vi "send&receive_TestSuite.vi"() -> ()   [LabVIEW 2018, in "LV2Julia_examples.lvlib"]
uses:
  LV2Julia_examples.lvlib
  LV2Julia_core/VIs/Server or client state.ctl
  LV2Julia_core/VIs/detailed error info.ctl
  LV2Julia_core/VIs/StackFrame.ctl
  LV2Julia_core/VIs/Numeric Types enum.ctl
  LV2Julia_core/VIs/Commands.ctl
  LV2Julia_core/VIs/commands LV2Jl.ctl
  0f3c6ff9-6efb-4048-9743-f0faf74ba571.vi
  a0325a13-fabe-4ce2-9e5f-cb47086c548e.vi
  7f01987e-74d6-4a03-8747-02f9f83a463d.vi
  79db7e0a-da4c-4117-a634-db979a193aea.vi
  99f1ef0e-755f-4741-8b5d-28859cadfccc.vi
  28f6b6a8-06e1-472c-a07e-67bcf9cc4e65.vi
  f8b325f9-9a1a-4df1-afd8-c5f3d250536f.vi
  a48dd356-bbba-47e0-9e2d-40331a29731c.vi
  80a357a5-d281-45e5-bb39-cf6b9d5a1e33.vi
  f79ed0ed-9efb-49b8-8cfa-ee86261ff89e.vi
  9cb09b36-286d-49e3-8dd2-a7b0f5b1e9d8.vi
  1a7f9d96-89a5-4905-829b-2a4edb26e723.vi
  cfafe85d-2515-4c22-937f-8121ed6e9d54.vi
  d2cb43a9-9305-42fb-ad58-bce983510195.vi
  0f3c6ff9-6efb-4048-9743-f0faf74ba571.vi/c050a881-ebb0-4e81-b48e-5d54ac6d298c.vi
  0f3c6ff9-6efb-4048-9743-f0faf74ba571.vi/f138d779-8015-4f82-8c48-da5c27a321f7.vi
  0f3c6ff9-6efb-4048-9743-f0faf74ba571.vi/6f5853da-1522-42ed-a631-8137277f6bd0.vi
  0f3c6ff9-6efb-4048-9743-f0faf74ba571.vi/334a13bf-ed79-421d-8f9d-442316ab956b.vi
  0f3c6ff9-6efb-4048-9743-f0faf74ba571.vi/8f08bb46-79c7-4cf6-8c43-e5292f35a42a.vi
  a0325a13-fabe-4ce2-9e5f-cb47086c548e.vi/0a023b70-b2b7-4b51-b4a8-1637e8f72752.vi
  a0325a13-fabe-4ce2-9e5f-cb47086c548e.vi/abfddf90-bad1-40a2-8341-74545abc888a.vi
  a0325a13-fabe-4ce2-9e5f-cb47086c548e.vi/e109d5e2-aea3-4de8-91e8-3aff7ff5e1a5.vi
  a0325a13-fabe-4ce2-9e5f-cb47086c548e.vi/2119aad2-e76b-4395-bc38-e2441a866829.vi
  a0325a13-fabe-4ce2-9e5f-cb47086c548e.vi/bbe2ee9c-aeb3-4e4f-93f8-3db8855d79ac.vi
  7f01987e-74d6-4a03-8747-02f9f83a463d.vi/bf06bc0c-d54c-4899-bc86-944563b4b303.vi
  7f01987e-74d6-4a03-8747-02f9f83a463d.vi/d4eb1beb-9046-40bb-82cb-9c8078805344.vi
  7f01987e-74d6-4a03-8747-02f9f83a463d.vi/5686e550-6946-4fb3-9876-dc3418ab0293.vi
  7f01987e-74d6-4a03-8747-02f9f83a463d.vi/ffdc1569-392d-4031-a554-eaded28feac0.vi
  7f01987e-74d6-4a03-8747-02f9f83a463d.vi/e28b746a-5d22-4361-bc60-6e965f2af8e6.vi
  79db7e0a-da4c-4117-a634-db979a193aea.vi/5c498217-6613-458c-8874-fa92d6c19748.vi
  79db7e0a-da4c-4117-a634-db979a193aea.vi/90651d55-7251-4542-bf1a-96215a5cb46c.vi
  79db7e0a-da4c-4117-a634-db979a193aea.vi/4ea0e9b0-802e-4012-92bd-3a6280912451.vi
  99f1ef0e-755f-4741-8b5d-28859cadfccc.vi/ccb71516-df13-49fa-b0f6-e0b8672de1da.vi
  99f1ef0e-755f-4741-8b5d-28859cadfccc.vi/34444bcf-5933-4351-bbc5-1eae9a0680b0.vi
  99f1ef0e-755f-4741-8b5d-28859cadfccc.vi/000cc600-1167-4cf4-928d-6ab7aa667d42.vi
  99f1ef0e-755f-4741-8b5d-28859cadfccc.vi/98e98eea-062a-4f87-a790-41d557d372ce.vi
  99f1ef0e-755f-4741-8b5d-28859cadfccc.vi/eb945e44-4973-4a99-b8fc-568457e51597.vi
  28f6b6a8-06e1-472c-a07e-67bcf9cc4e65.vi/09974be2-1a4f-442e-861e-99198c07ad3e.vi
  28f6b6a8-06e1-472c-a07e-67bcf9cc4e65.vi/d0db5e8f-3a3c-4f1f-98d6-975ebc25a533.vi
  28f6b6a8-06e1-472c-a07e-67bcf9cc4e65.vi/c2a43064-5d3e-4f07-a41e-f48ba3bb7a5d.vi
  28f6b6a8-06e1-472c-a07e-67bcf9cc4e65.vi/cb57ac50-2f4d-40c6-84c3-4b337ccbba5c.vi
  28f6b6a8-06e1-472c-a07e-67bcf9cc4e65.vi/ce760082-6063-416a-be6f-af541c50d0f9.vi
  f8b325f9-9a1a-4df1-afd8-c5f3d250536f.vi/d0a21f22-daf0-459d-8dea-c9de37d976a3.vi
  f8b325f9-9a1a-4df1-afd8-c5f3d250536f.vi/3938edcc-9689-4aa2-8890-51d0be5f89a6.vi
  f8b325f9-9a1a-4df1-afd8-c5f3d250536f.vi/ea9f557a-cbf4-4eb9-9afd-8566b7af0bf0.vi
  f8b325f9-9a1a-4df1-afd8-c5f3d250536f.vi/f50092b0-9f6c-4b67-b069-c79229ff8c92.vi
  f8b325f9-9a1a-4df1-afd8-c5f3d250536f.vi/d586cd56-0096-4f37-b8fb-3a75e4053398.vi
  a48dd356-bbba-47e0-9e2d-40331a29731c.vi/60485b63-9fa3-41d8-b025-f222c2d1e954.vi
  a48dd356-bbba-47e0-9e2d-40331a29731c.vi/0163ca4a-c9bf-4356-9374-5b2f1cd8c8a4.vi
  a48dd356-bbba-47e0-9e2d-40331a29731c.vi/cdf03f06-3cc5-4344-93be-09e3c2b5fad7.vi
  a48dd356-bbba-47e0-9e2d-40331a29731c.vi/9e91637f-31fa-49b3-9c25-505779283418.vi
  a48dd356-bbba-47e0-9e2d-40331a29731c.vi/a6edc50e-f715-450b-aaf1-fcba25539407.vi
  80a357a5-d281-45e5-bb39-cf6b9d5a1e33.vi/4a5881ab-1715-4bbe-9af8-2363ce582ba4.vi
  80a357a5-d281-45e5-bb39-cf6b9d5a1e33.vi/b95eb402-4789-4c76-85b7-fbdb598d54ac.vi
  80a357a5-d281-45e5-bb39-cf6b9d5a1e33.vi/1290ab50-9fc8-4350-9e5d-3eaedcb8adb4.vi
  80a357a5-d281-45e5-bb39-cf6b9d5a1e33.vi/25ba802a-e149-482c-ab2a-a4ec831a7ccd.vi
  80a357a5-d281-45e5-bb39-cf6b9d5a1e33.vi/46001291-25fa-4f3c-9091-6cb6f22db868.vi
  f79ed0ed-9efb-49b8-8cfa-ee86261ff89e.vi/3667ecba-1e4f-48f0-93f6-750241537af3.vi
  f79ed0ed-9efb-49b8-8cfa-ee86261ff89e.vi/099a3fa0-6d4e-42af-8655-f73d0e4a363a.vi
  f79ed0ed-9efb-49b8-8cfa-ee86261ff89e.vi/1be80b05-b2d8-4daf-8502-32be035b1a56.vi
  f79ed0ed-9efb-49b8-8cfa-ee86261ff89e.vi/01dbd68c-7ff6-4de3-9551-88d27b9349fc.vi
  f79ed0ed-9efb-49b8-8cfa-ee86261ff89e.vi/d0bca59b-d26b-4ea8-bc33-01712e7e045f.vi
  9cb09b36-286d-49e3-8dd2-a7b0f5b1e9d8.vi/cfaefed5-3f29-4c43-88dd-88c8fc82987c.vi
  9cb09b36-286d-49e3-8dd2-a7b0f5b1e9d8.vi/62ff6e0a-46cc-460d-9e84-467dd4467122.vi
  9cb09b36-286d-49e3-8dd2-a7b0f5b1e9d8.vi/bc301213-06cb-494c-a645-9c5eb5ccddf2.vi
  9cb09b36-286d-49e3-8dd2-a7b0f5b1e9d8.vi/e85f0252-b661-475b-8e20-7d78206805a9.vi
  9cb09b36-286d-49e3-8dd2-a7b0f5b1e9d8.vi/e3c6487d-5533-439a-972b-ff6e78f91a0f.vi
  1a7f9d96-89a5-4905-829b-2a4edb26e723.vi/057b0a30-89eb-4b99-9a94-261e0d1b69db.vi
  1a7f9d96-89a5-4905-829b-2a4edb26e723.vi/1be28d80-beb7-4371-90e4-946dee281c8c.vi
  1a7f9d96-89a5-4905-829b-2a4edb26e723.vi/3a062081-cf3a-4e63-a10a-adcd83a17c12.vi
  1a7f9d96-89a5-4905-829b-2a4edb26e723.vi/70040952-3ae0-468b-bc38-5f997367fd6f.vi
  1a7f9d96-89a5-4905-829b-2a4edb26e723.vi/69db4b1a-60c2-40fd-b347-670db0906532.vi
  cfafe85d-2515-4c22-937f-8121ed6e9d54.vi/9bad1c1b-63c8-4bce-9a14-6c192ddbd00b.vi
  cfafe85d-2515-4c22-937f-8121ed6e9d54.vi/11fa2f37-74a1-4205-9996-7863193281ff.vi
  cfafe85d-2515-4c22-937f-8121ed6e9d54.vi/07d86764-f698-4878-be38-d6e095ca1645.vi
  cfafe85d-2515-4c22-937f-8121ed6e9d54.vi/c0e3ea08-1ccb-4dcb-b733-8d3fe66c5f6f.vi
  cfafe85d-2515-4c22-937f-8121ed6e9d54.vi/1336a158-84d5-45d6-a2b2-5b90658c6328.vi
  d2cb43a9-9305-42fb-ad58-bce983510195.vi/18912dc4-b1e0-4230-8a87-9373dc369598.vi
  d2cb43a9-9305-42fb-ad58-bce983510195.vi/6312c1e7-5e2e-4310-bd4a-23119c15d3f1.vi
  d2cb43a9-9305-42fb-ad58-bce983510195.vi/9cb92e57-85ab-440f-a46b-8557216ab5dd.vi
  0f3c6ff9-6efb-4048-9743-f0faf74ba571.vi/f138d779-8015-4f82-8c48-da5c27a321f7.vi/dcaca655-459b-49bd-b29b-dd229471a558.vi
  0f3c6ff9-6efb-4048-9743-f0faf74ba571.vi/6f5853da-1522-42ed-a631-8137277f6bd0.vi/6ca8c9a2-308c-4824-adeb-58a98f4b9789.vi
  0f3c6ff9-6efb-4048-9743-f0faf74ba571.vi/334a13bf-ed79-421d-8f9d-442316ab956b.vi/c3e25d4f-3d6e-45b4-ac60-a3eac4f5d4dd.vi
  a0325a13-fabe-4ce2-9e5f-cb47086c548e.vi/abfddf90-bad1-40a2-8341-74545abc888a.vi/1d4ccc36-5df4-463a-a9dd-e871d8c5e836.vi
  a0325a13-fabe-4ce2-9e5f-cb47086c548e.vi/e109d5e2-aea3-4de8-91e8-3aff7ff5e1a5.vi/72ea6f5e-8e76-457b-9f2b-3a011e948c95.vi
  a0325a13-fabe-4ce2-9e5f-cb47086c548e.vi/2119aad2-e76b-4395-bc38-e2441a866829.vi/a15880f2-4104-4f97-a4bf-5a36a63c211d.vi
  7f01987e-74d6-4a03-8747-02f9f83a463d.vi/d4eb1beb-9046-40bb-82cb-9c8078805344.vi/f0e9f2d5-ddd8-4b96-91ce-de174306b7a9.vi
  7f01987e-74d6-4a03-8747-02f9f83a463d.vi/5686e550-6946-4fb3-9876-dc3418ab0293.vi/45224409-fc74-4a19-bc5d-04c35b5f3d3a.vi
  7f01987e-74d6-4a03-8747-02f9f83a463d.vi/ffdc1569-392d-4031-a554-eaded28feac0.vi/9cbce8f5-06a0-437b-b659-713dc5751795.vi
  79db7e0a-da4c-4117-a634-db979a193aea.vi/5c498217-6613-458c-8874-fa92d6c19748.vi/0922e35c-3983-4244-89a6-de18eb35483c.vi
  79db7e0a-da4c-4117-a634-db979a193aea.vi/90651d55-7251-4542-bf1a-96215a5cb46c.vi/23ce4379-b224-4a09-8a60-6986842fc155.vi
  79db7e0a-da4c-4117-a634-db979a193aea.vi/4ea0e9b0-802e-4012-92bd-3a6280912451.vi/5cb0fd22-39b3-4679-8848-fbd0f76a760c.vi
  99f1ef0e-755f-4741-8b5d-28859cadfccc.vi/34444bcf-5933-4351-bbc5-1eae9a0680b0.vi/9b5ee3b2-61fa-464d-b808-4ed852ba9df7.vi
  99f1ef0e-755f-4741-8b5d-28859cadfccc.vi/000cc600-1167-4cf4-928d-6ab7aa667d42.vi/729371f3-82b8-4148-8e0c-782b1393dd88.vi
  99f1ef0e-755f-4741-8b5d-28859cadfccc.vi/98e98eea-062a-4f87-a790-41d557d372ce.vi/7cea73a9-e450-4982-a850-64259969e5c4.vi
  28f6b6a8-06e1-472c-a07e-67bcf9cc4e65.vi/d0db5e8f-3a3c-4f1f-98d6-975ebc25a533.vi/c32e5faa-0551-4674-b326-206195be28cb.vi
  28f6b6a8-06e1-472c-a07e-67bcf9cc4e65.vi/c2a43064-5d3e-4f07-a41e-f48ba3bb7a5d.vi/b2b31e85-ff8a-4a11-b6da-4397c20cf58c.vi
  28f6b6a8-06e1-472c-a07e-67bcf9cc4e65.vi/cb57ac50-2f4d-40c6-84c3-4b337ccbba5c.vi/00287ef4-4dad-445f-b53f-6d398869e1f1.vi
  f8b325f9-9a1a-4df1-afd8-c5f3d250536f.vi/3938edcc-9689-4aa2-8890-51d0be5f89a6.vi/9b496619-56e3-46e5-9420-f0b2b562818d.vi
  f8b325f9-9a1a-4df1-afd8-c5f3d250536f.vi/ea9f557a-cbf4-4eb9-9afd-8566b7af0bf0.vi/c59bfabf-8824-4878-9e47-809c29df3a14.vi
  f8b325f9-9a1a-4df1-afd8-c5f3d250536f.vi/f50092b0-9f6c-4b67-b069-c79229ff8c92.vi/f21eb179-c848-459d-95dc-6ea7d11ae3e0.vi
  a48dd356-bbba-47e0-9e2d-40331a29731c.vi/0163ca4a-c9bf-4356-9374-5b2f1cd8c8a4.vi/d72399aa-8d74-4fbe-b140-3f7c8dcdc190.vi
  a48dd356-bbba-47e0-9e2d-40331a29731c.vi/cdf03f06-3cc5-4344-93be-09e3c2b5fad7.vi/030a484a-d102-49b4-9b08-46c7516c605d.vi
  a48dd356-bbba-47e0-9e2d-40331a29731c.vi/9e91637f-31fa-49b3-9c25-505779283418.vi/50726ecf-c9f1-4d31-8d96-37015bd9bd52.vi
  80a357a5-d281-45e5-bb39-cf6b9d5a1e33.vi/b95eb402-4789-4c76-85b7-fbdb598d54ac.vi/a5383ccf-8e63-4c19-8ea6-c4f731bf680f.vi
  80a357a5-d281-45e5-bb39-cf6b9d5a1e33.vi/1290ab50-9fc8-4350-9e5d-3eaedcb8adb4.vi/8e8fe23a-c37e-4fb9-bc35-54979b00683a.vi
  80a357a5-d281-45e5-bb39-cf6b9d5a1e33.vi/25ba802a-e149-482c-ab2a-a4ec831a7ccd.vi/f1769c1e-122f-4ecb-91b4-8a90a66d4ed8.vi
  f79ed0ed-9efb-49b8-8cfa-ee86261ff89e.vi/099a3fa0-6d4e-42af-8655-f73d0e4a363a.vi/8ccb3943-b745-4649-895e-cc58cd628f04.vi
  f79ed0ed-9efb-49b8-8cfa-ee86261ff89e.vi/1be80b05-b2d8-4daf-8502-32be035b1a56.vi/9ebaa59b-334c-4cc3-a2e7-5942a76866e6.vi
  f79ed0ed-9efb-49b8-8cfa-ee86261ff89e.vi/01dbd68c-7ff6-4de3-9551-88d27b9349fc.vi/70455b90-e97b-459b-985c-d87a1c5f8d27.vi
  9cb09b36-286d-49e3-8dd2-a7b0f5b1e9d8.vi/62ff6e0a-46cc-460d-9e84-467dd4467122.vi/df185cf5-c5c8-4528-bf4e-04034ca71658.vi
  9cb09b36-286d-49e3-8dd2-a7b0f5b1e9d8.vi/bc301213-06cb-494c-a645-9c5eb5ccddf2.vi/68ecb473-ff7a-4f33-a7f5-8ddef986aaf0.vi
  9cb09b36-286d-49e3-8dd2-a7b0f5b1e9d8.vi/e85f0252-b661-475b-8e20-7d78206805a9.vi/805f8906-2ac2-4943-bcc2-ce7ee6626e70.vi
  1a7f9d96-89a5-4905-829b-2a4edb26e723.vi/1be28d80-beb7-4371-90e4-946dee281c8c.vi/29c07661-3584-43cb-8413-0ad855bf1dd6.vi
  1a7f9d96-89a5-4905-829b-2a4edb26e723.vi/3a062081-cf3a-4e63-a10a-adcd83a17c12.vi/92de0394-8b0e-41a9-bbdb-0ba419639912.vi
  1a7f9d96-89a5-4905-829b-2a4edb26e723.vi/70040952-3ae0-468b-bc38-5f997367fd6f.vi/85e2adf1-435c-4f2b-9704-a4fe5359d41d.vi
  cfafe85d-2515-4c22-937f-8121ed6e9d54.vi/11fa2f37-74a1-4205-9996-7863193281ff.vi/e77d8312-4832-4633-a75f-e330979cf09b.vi
  cfafe85d-2515-4c22-937f-8121ed6e9d54.vi/07d86764-f698-4878-be38-d6e095ca1645.vi/c76a7bcb-882a-45a4-b89f-2597d2f33847.vi
  cfafe85d-2515-4c22-937f-8121ed6e9d54.vi/c0e3ea08-1ccb-4dcb-b733-8d3fe66c5f6f.vi/c3839c05-a494-4270-b8a7-0c53a6508c74.vi
  0f3c6ff9-6efb-4048-9743-f0faf74ba571.vi/f138d779-8015-4f82-8c48-da5c27a321f7.vi/dcaca655-459b-49bd-b29b-dd229471a558.vi/2309c166-be4b-4e1e-8eb3-967cc5e528c7.vi
  0f3c6ff9-6efb-4048-9743-f0faf74ba571.vi/6f5853da-1522-42ed-a631-8137277f6bd0.vi/6ca8c9a2-308c-4824-adeb-58a98f4b9789.vi/cc0f1ca1-4239-4878-a66c-6570c0dfb283.vi
  0f3c6ff9-6efb-4048-9743-f0faf74ba571.vi/334a13bf-ed79-421d-8f9d-442316ab956b.vi/c3e25d4f-3d6e-45b4-ac60-a3eac4f5d4dd.vi/ab71de19-15ae-471d-8a17-25537f6b9f7d.vi
  a0325a13-fabe-4ce2-9e5f-cb47086c548e.vi/abfddf90-bad1-40a2-8341-74545abc888a.vi/1d4ccc36-5df4-463a-a9dd-e871d8c5e836.vi/621a2642-8e80-4bc6-8a7b-f91475f6563b.vi
  a0325a13-fabe-4ce2-9e5f-cb47086c548e.vi/e109d5e2-aea3-4de8-91e8-3aff7ff5e1a5.vi/72ea6f5e-8e76-457b-9f2b-3a011e948c95.vi/d84d9467-773a-4f51-b374-34f3b45e96f8.vi
  a0325a13-fabe-4ce2-9e5f-cb47086c548e.vi/2119aad2-e76b-4395-bc38-e2441a866829.vi/a15880f2-4104-4f97-a4bf-5a36a63c211d.vi/9e7459c3-f81a-4fcd-bf47-d21a6f8ffe87.vi
  7f01987e-74d6-4a03-8747-02f9f83a463d.vi/d4eb1beb-9046-40bb-82cb-9c8078805344.vi/f0e9f2d5-ddd8-4b96-91ce-de174306b7a9.vi/6f36de78-967c-4933-b5dd-0e598d4ad331.vi
  7f01987e-74d6-4a03-8747-02f9f83a463d.vi/5686e550-6946-4fb3-9876-dc3418ab0293.vi/45224409-fc74-4a19-bc5d-04c35b5f3d3a.vi/c4da7d02-ca8d-4870-8b8b-0b3c510ded96.vi
  7f01987e-74d6-4a03-8747-02f9f83a463d.vi/ffdc1569-392d-4031-a554-eaded28feac0.vi/9cbce8f5-06a0-437b-b659-713dc5751795.vi/16954a76-b9b0-4a64-9d17-38344290d572.vi
  79db7e0a-da4c-4117-a634-db979a193aea.vi/5c498217-6613-458c-8874-fa92d6c19748.vi/0922e35c-3983-4244-89a6-de18eb35483c.vi/42b4f21c-8679-4e81-9200-b8334ca139f1.vi
  79db7e0a-da4c-4117-a634-db979a193aea.vi/90651d55-7251-4542-bf1a-96215a5cb46c.vi/23ce4379-b224-4a09-8a60-6986842fc155.vi/1d0a4c10-6ff0-4457-9a73-6ff640e2168e.vi
  79db7e0a-da4c-4117-a634-db979a193aea.vi/4ea0e9b0-802e-4012-92bd-3a6280912451.vi/5cb0fd22-39b3-4679-8848-fbd0f76a760c.vi/38b5f270-5c40-4c58-9d4f-444c3803379d.vi
  99f1ef0e-755f-4741-8b5d-28859cadfccc.vi/34444bcf-5933-4351-bbc5-1eae9a0680b0.vi/9b5ee3b2-61fa-464d-b808-4ed852ba9df7.vi/79d9312b-1957-4e85-8002-522c7c56894f.vi
  99f1ef0e-755f-4741-8b5d-28859cadfccc.vi/000cc600-1167-4cf4-928d-6ab7aa667d42.vi/729371f3-82b8-4148-8e0c-782b1393dd88.vi/94117fd3-7e95-4c61-9d4c-d51d7f218b0b.vi
  99f1ef0e-755f-4741-8b5d-28859cadfccc.vi/98e98eea-062a-4f87-a790-41d557d372ce.vi/7cea73a9-e450-4982-a850-64259969e5c4.vi/fdf70d00-e57a-4a1e-bdd4-d33344dbcdc5.vi
  28f6b6a8-06e1-472c-a07e-67bcf9cc4e65.vi/d0db5e8f-3a3c-4f1f-98d6-975ebc25a533.vi/c32e5faa-0551-4674-b326-206195be28cb.vi/0d0755cb-849f-424c-b832-95ef875b3293.vi
  28f6b6a8-06e1-472c-a07e-67bcf9cc4e65.vi/c2a43064-5d3e-4f07-a41e-f48ba3bb7a5d.vi/b2b31e85-ff8a-4a11-b6da-4397c20cf58c.vi/5bc3ebd1-2eea-4fe2-bd89-161902e93dbd.vi
  28f6b6a8-06e1-472c-a07e-67bcf9cc4e65.vi/cb57ac50-2f4d-40c6-84c3-4b337ccbba5c.vi/00287ef4-4dad-445f-b53f-6d398869e1f1.vi/604b13c5-3f03-4950-a4a6-8625370b5ea2.vi
  f8b325f9-9a1a-4df1-afd8-c5f3d250536f.vi/3938edcc-9689-4aa2-8890-51d0be5f89a6.vi/9b496619-56e3-46e5-9420-f0b2b562818d.vi/5740d471-efac-432f-8db3-bced88e252bb.vi
  f8b325f9-9a1a-4df1-afd8-c5f3d250536f.vi/ea9f557a-cbf4-4eb9-9afd-8566b7af0bf0.vi/c59bfabf-8824-4878-9e47-809c29df3a14.vi/6a753862-9d09-495d-b4f7-b2d74518f4a9.vi
  f8b325f9-9a1a-4df1-afd8-c5f3d250536f.vi/f50092b0-9f6c-4b67-b069-c79229ff8c92.vi/f21eb179-c848-459d-95dc-6ea7d11ae3e0.vi/f4d8b248-fa08-4394-b4bf-415efba63cb6.vi
  a48dd356-bbba-47e0-9e2d-40331a29731c.vi/0163ca4a-c9bf-4356-9374-5b2f1cd8c8a4.vi/d72399aa-8d74-4fbe-b140-3f7c8dcdc190.vi/704d183b-2037-459a-ade8-6df426d2bfbd.vi
  a48dd356-bbba-47e0-9e2d-40331a29731c.vi/cdf03f06-3cc5-4344-93be-09e3c2b5fad7.vi/030a484a-d102-49b4-9b08-46c7516c605d.vi/6afecd3f-41c9-48e9-a420-169fc65296cf.vi
  a48dd356-bbba-47e0-9e2d-40331a29731c.vi/9e91637f-31fa-49b3-9c25-505779283418.vi/50726ecf-c9f1-4d31-8d96-37015bd9bd52.vi/84b9b7d2-2a4f-4508-b6a4-45f87f7c3a5d.vi
  80a357a5-d281-45e5-bb39-cf6b9d5a1e33.vi/b95eb402-4789-4c76-85b7-fbdb598d54ac.vi/a5383ccf-8e63-4c19-8ea6-c4f731bf680f.vi/7a3d23f4-78d6-428f-aabb-d22b9a7765ad.vi
  80a357a5-d281-45e5-bb39-cf6b9d5a1e33.vi/1290ab50-9fc8-4350-9e5d-3eaedcb8adb4.vi/8e8fe23a-c37e-4fb9-bc35-54979b00683a.vi/8fc8ec74-8d15-4e22-bb13-3bab23306641.vi
  80a357a5-d281-45e5-bb39-cf6b9d5a1e33.vi/25ba802a-e149-482c-ab2a-a4ec831a7ccd.vi/f1769c1e-122f-4ecb-91b4-8a90a66d4ed8.vi/a6480028-143d-449f-a90d-1715e38a0322.vi
  f79ed0ed-9efb-49b8-8cfa-ee86261ff89e.vi/099a3fa0-6d4e-42af-8655-f73d0e4a363a.vi/8ccb3943-b745-4649-895e-cc58cd628f04.vi/91ad8c32-2595-463f-a00d-19f1a31a0ab9.vi
  f79ed0ed-9efb-49b8-8cfa-ee86261ff89e.vi/1be80b05-b2d8-4daf-8502-32be035b1a56.vi/9ebaa59b-334c-4cc3-a2e7-5942a76866e6.vi/d7ca76aa-8f91-40c8-a33d-e0fc436d8429.vi
  f79ed0ed-9efb-49b8-8cfa-ee86261ff89e.vi/01dbd68c-7ff6-4de3-9551-88d27b9349fc.vi/70455b90-e97b-459b-985c-d87a1c5f8d27.vi/8334b92e-6c89-421a-9a89-9393042ee175.vi
  9cb09b36-286d-49e3-8dd2-a7b0f5b1e9d8.vi/62ff6e0a-46cc-460d-9e84-467dd4467122.vi/df185cf5-c5c8-4528-bf4e-04034ca71658.vi/555e92da-38c3-4728-ae1a-7d35d47cec6d.vi
  9cb09b36-286d-49e3-8dd2-a7b0f5b1e9d8.vi/bc301213-06cb-494c-a645-9c5eb5ccddf2.vi/68ecb473-ff7a-4f33-a7f5-8ddef986aaf0.vi/2cb7f626-0a6b-40e1-a36b-1fffb410bdb6.vi
  9cb09b36-286d-49e3-8dd2-a7b0f5b1e9d8.vi/e85f0252-b661-475b-8e20-7d78206805a9.vi/805f8906-2ac2-4943-bcc2-ce7ee6626e70.vi/1a5fcff8-1e1b-4a10-8cb0-04266a3492f5.vi
  1a7f9d96-89a5-4905-829b-2a4edb26e723.vi/1be28d80-beb7-4371-90e4-946dee281c8c.vi/29c07661-3584-43cb-8413-0ad855bf1dd6.vi/274c10cc-6877-4fb6-876e-52686d1825c0.vi
  1a7f9d96-89a5-4905-829b-2a4edb26e723.vi/3a062081-cf3a-4e63-a10a-adcd83a17c12.vi/92de0394-8b0e-41a9-bbdb-0ba419639912.vi/ec3eeeb6-efa3-447e-bef4-ff225729b20e.vi
  1a7f9d96-89a5-4905-829b-2a4edb26e723.vi/70040952-3ae0-468b-bc38-5f997367fd6f.vi/85e2adf1-435c-4f2b-9704-a4fe5359d41d.vi/53a65439-65bc-4240-a9ef-cc811b2bd780.vi
  cfafe85d-2515-4c22-937f-8121ed6e9d54.vi/11fa2f37-74a1-4205-9996-7863193281ff.vi/e77d8312-4832-4633-a75f-e330979cf09b.vi/aed36081-aed2-409f-bc39-66819cd0b4c3.vi
  cfafe85d-2515-4c22-937f-8121ed6e9d54.vi/07d86764-f698-4878-be38-d6e095ca1645.vi/c76a7bcb-882a-45a4-b89f-2597d2f33847.vi/54c288f8-840e-43b8-aaff-0bb173d43f54.vi
  cfafe85d-2515-4c22-937f-8121ed6e9d54.vi/c0e3ea08-1ccb-4dcb-b733-8d3fe66c5f6f.vi/c3839c05-a494-4270-b8a7-0c53a6508c74.vi/3cadb2ed-87ca-4814-8e99-a2e720a8dfb1.vi
  0f3c6ff9-6efb-4048-9743-f0faf74ba571.vi/f138d779-8015-4f82-8c48-da5c27a321f7.vi/dcaca655-459b-49bd-b29b-dd229471a558.vi/2309c166-be4b-4e1e-8eb3-967cc5e528c7.vi/f6d3542d-cc1e-4d9d-9817-8d6bc396b8a7.vi
  0f3c6ff9-6efb-4048-9743-f0faf74ba571.vi/6f5853da-1522-42ed-a631-8137277f6bd0.vi/6ca8c9a2-308c-4824-adeb-58a98f4b9789.vi/cc0f1ca1-4239-4878-a66c-6570c0dfb283.vi/ff7285a8-522c-43fc-9d63-dac79a8fad90.vi
  0f3c6ff9-6efb-4048-9743-f0faf74ba571.vi/334a13bf-ed79-421d-8f9d-442316ab956b.vi/c3e25d4f-3d6e-45b4-ac60-a3eac4f5d4dd.vi/ab71de19-15ae-471d-8a17-25537f6b9f7d.vi/091f02b8-9279-4536-a74d-e36162d3ff9a.vi
  a0325a13-fabe-4ce2-9e5f-cb47086c548e.vi/abfddf90-bad1-40a2-8341-74545abc888a.vi/1d4ccc36-5df4-463a-a9dd-e871d8c5e836.vi/621a2642-8e80-4bc6-8a7b-f91475f6563b.vi/f9b6ac16-1dbf-42f9-a70d-5fd8ed98ba9f.vi
  a0325a13-fabe-4ce2-9e5f-cb47086c548e.vi/e109d5e2-aea3-4de8-91e8-3aff7ff5e1a5.vi/72ea6f5e-8e76-457b-9f2b-3a011e948c95.vi/d84d9467-773a-4f51-b374-34f3b45e96f8.vi/1fa9ed59-771e-41ed-bb50-82ff1c775e4b.vi
  a0325a13-fabe-4ce2-9e5f-cb47086c548e.vi/2119aad2-e76b-4395-bc38-e2441a866829.vi/a15880f2-4104-4f97-a4bf-5a36a63c211d.vi/9e7459c3-f81a-4fcd-bf47-d21a6f8ffe87.vi/04f1935c-411d-4607-b276-13542326c360.vi
  7f01987e-74d6-4a03-8747-02f9f83a463d.vi/d4eb1beb-9046-40bb-82cb-9c8078805344.vi/f0e9f2d5-ddd8-4b96-91ce-de174306b7a9.vi/6f36de78-967c-4933-b5dd-0e598d4ad331.vi/3483b618-6941-450d-853a-3dd4f80d8194.vi
  7f01987e-74d6-4a03-8747-02f9f83a463d.vi/5686e550-6946-4fb3-9876-dc3418ab0293.vi/45224409-fc74-4a19-bc5d-04c35b5f3d3a.vi/c4da7d02-ca8d-4870-8b8b-0b3c510ded96.vi/369bf8c1-16ba-47de-918f-01b187e51fbd.vi
  7f01987e-74d6-4a03-8747-02f9f83a463d.vi/ffdc1569-392d-4031-a554-eaded28feac0.vi/9cbce8f5-06a0-437b-b659-713dc5751795.vi/16954a76-b9b0-4a64-9d17-38344290d572.vi/b76e1231-7917-4139-a770-2dbef96067c6.vi
  79db7e0a-da4c-4117-a634-db979a193aea.vi/5c498217-6613-458c-8874-fa92d6c19748.vi/0922e35c-3983-4244-89a6-de18eb35483c.vi/42b4f21c-8679-4e81-9200-b8334ca139f1.vi/cdd67d70-fed5-40eb-bd55-64c7d9f8c0cd.vi
  79db7e0a-da4c-4117-a634-db979a193aea.vi/90651d55-7251-4542-bf1a-96215a5cb46c.vi/23ce4379-b224-4a09-8a60-6986842fc155.vi/1d0a4c10-6ff0-4457-9a73-6ff640e2168e.vi/b5e6a49d-e123-41cd-ae39-6a04b1010118.vi
  79db7e0a-da4c-4117-a634-db979a193aea.vi/4ea0e9b0-802e-4012-92bd-3a6280912451.vi/5cb0fd22-39b3-4679-8848-fbd0f76a760c.vi/38b5f270-5c40-4c58-9d4f-444c3803379d.vi/80dd6213-b969-49b8-828d-e6a134ffc038.vi
  99f1ef0e-755f-4741-8b5d-28859cadfccc.vi/34444bcf-5933-4351-bbc5-1eae9a0680b0.vi/9b5ee3b2-61fa-464d-b808-4ed852ba9df7.vi/79d9312b-1957-4e85-8002-522c7c56894f.vi/63dab871-5128-418b-a9d4-6181b1149ad7.vi
  99f1ef0e-755f-4741-8b5d-28859cadfccc.vi/000cc600-1167-4cf4-928d-6ab7aa667d42.vi/729371f3-82b8-4148-8e0c-782b1393dd88.vi/94117fd3-7e95-4c61-9d4c-d51d7f218b0b.vi/69c89fbf-0cd2-4258-9685-0a42dcae2355.vi
  99f1ef0e-755f-4741-8b5d-28859cadfccc.vi/98e98eea-062a-4f87-a790-41d557d372ce.vi/7cea73a9-e450-4982-a850-64259969e5c4.vi/fdf70d00-e57a-4a1e-bdd4-d33344dbcdc5.vi/a0095e46-2272-4885-97f1-c4be5742910c.vi
  28f6b6a8-06e1-472c-a07e-67bcf9cc4e65.vi/d0db5e8f-3a3c-4f1f-98d6-975ebc25a533.vi/c32e5faa-0551-4674-b326-206195be28cb.vi/0d0755cb-849f-424c-b832-95ef875b3293.vi/4bf715f5-e116-42cd-bc7a-13d076c33e15.vi
  28f6b6a8-06e1-472c-a07e-67bcf9cc4e65.vi/c2a43064-5d3e-4f07-a41e-f48ba3bb7a5d.vi/b2b31e85-ff8a-4a11-b6da-4397c20cf58c.vi/5bc3ebd1-2eea-4fe2-bd89-161902e93dbd.vi/b8763943-8b18-49e5-bcd9-5f6519a8b2c5.vi
  28f6b6a8-06e1-472c-a07e-67bcf9cc4e65.vi/cb57ac50-2f4d-40c6-84c3-4b337ccbba5c.vi/00287ef4-4dad-445f-b53f-6d398869e1f1.vi/604b13c5-3f03-4950-a4a6-8625370b5ea2.vi/1fd5b09f-ec90-4e67-91ff-e84f89ca8c25.vi
  f8b325f9-9a1a-4df1-afd8-c5f3d250536f.vi/3938edcc-9689-4aa2-8890-51d0be5f89a6.vi/9b496619-56e3-46e5-9420-f0b2b562818d.vi/5740d471-efac-432f-8db3-bced88e252bb.vi/9f0b073e-b391-4280-a90c-85d02cefbfb1.vi
  f8b325f9-9a1a-4df1-afd8-c5f3d250536f.vi/ea9f557a-cbf4-4eb9-9afd-8566b7af0bf0.vi/c59bfabf-8824-4878-9e47-809c29df3a14.vi/6a753862-9d09-495d-b4f7-b2d74518f4a9.vi/7897e5e8-eaa8-4330-bf23-fc2998fe9bb9.vi
  f8b325f9-9a1a-4df1-afd8-c5f3d250536f.vi/f50092b0-9f6c-4b67-b069-c79229ff8c92.vi/f21eb179-c848-459d-95dc-6ea7d11ae3e0.vi/f4d8b248-fa08-4394-b4bf-415efba63cb6.vi/8e058e81-a9b7-44e4-9997-a38aa5bfc02f.vi
  a48dd356-bbba-47e0-9e2d-40331a29731c.vi/0163ca4a-c9bf-4356-9374-5b2f1cd8c8a4.vi/d72399aa-8d74-4fbe-b140-3f7c8dcdc190.vi/704d183b-2037-459a-ade8-6df426d2bfbd.vi/289cce88-8c4c-435a-8e2c-a078df117b9e.vi
  a48dd356-bbba-47e0-9e2d-40331a29731c.vi/cdf03f06-3cc5-4344-93be-09e3c2b5fad7.vi/030a484a-d102-49b4-9b08-46c7516c605d.vi/6afecd3f-41c9-48e9-a420-169fc65296cf.vi/27de24e4-830a-48d0-a5fe-ff9ed3d4be87.vi
  a48dd356-bbba-47e0-9e2d-40331a29731c.vi/9e91637f-31fa-49b3-9c25-505779283418.vi/50726ecf-c9f1-4d31-8d96-37015bd9bd52.vi/84b9b7d2-2a4f-4508-b6a4-45f87f7c3a5d.vi/bc45bda0-d671-4435-853f-da6377ab6c0f.vi
  80a357a5-d281-45e5-bb39-cf6b9d5a1e33.vi/b95eb402-4789-4c76-85b7-fbdb598d54ac.vi/a5383ccf-8e63-4c19-8ea6-c4f731bf680f.vi/7a3d23f4-78d6-428f-aabb-d22b9a7765ad.vi/11c33436-193b-44c9-977d-ececd4a6ac51.vi
  80a357a5-d281-45e5-bb39-cf6b9d5a1e33.vi/1290ab50-9fc8-4350-9e5d-3eaedcb8adb4.vi/8e8fe23a-c37e-4fb9-bc35-54979b00683a.vi/8fc8ec74-8d15-4e22-bb13-3bab23306641.vi/f4fd83e8-1d8c-4823-9409-a0c4ae51a48c.vi
  80a357a5-d281-45e5-bb39-cf6b9d5a1e33.vi/25ba802a-e149-482c-ab2a-a4ec831a7ccd.vi/f1769c1e-122f-4ecb-91b4-8a90a66d4ed8.vi/a6480028-143d-449f-a90d-1715e38a0322.vi/99ca01ae-a83f-49a5-ae4a-080814a967d1.vi
  f79ed0ed-9efb-49b8-8cfa-ee86261ff89e.vi/099a3fa0-6d4e-42af-8655-f73d0e4a363a.vi/8ccb3943-b745-4649-895e-cc58cd628f04.vi/91ad8c32-2595-463f-a00d-19f1a31a0ab9.vi/0fc86a2f-760c-4000-a558-6625ae050d9c.vi
  f79ed0ed-9efb-49b8-8cfa-ee86261ff89e.vi/1be80b05-b2d8-4daf-8502-32be035b1a56.vi/9ebaa59b-334c-4cc3-a2e7-5942a76866e6.vi/d7ca76aa-8f91-40c8-a33d-e0fc436d8429.vi/a53a8712-ce2d-40f2-8719-5dedfc640ef9.vi
  f79ed0ed-9efb-49b8-8cfa-ee86261ff89e.vi/01dbd68c-7ff6-4de3-9551-88d27b9349fc.vi/70455b90-e97b-459b-985c-d87a1c5f8d27.vi/8334b92e-6c89-421a-9a89-9393042ee175.vi/474b7793-7654-4cc7-b10a-cc58eaf29e4f.vi
  9cb09b36-286d-49e3-8dd2-a7b0f5b1e9d8.vi/62ff6e0a-46cc-460d-9e84-467dd4467122.vi/df185cf5-c5c8-4528-bf4e-04034ca71658.vi/555e92da-38c3-4728-ae1a-7d35d47cec6d.vi/1ae85664-b332-44d4-867b-1d717d01f1b1.vi
  9cb09b36-286d-49e3-8dd2-a7b0f5b1e9d8.vi/bc301213-06cb-494c-a645-9c5eb5ccddf2.vi/68ecb473-ff7a-4f33-a7f5-8ddef986aaf0.vi/2cb7f626-0a6b-40e1-a36b-1fffb410bdb6.vi/525e6f11-a507-4ab5-8f44-f4f55daf67d4.vi
  9cb09b36-286d-49e3-8dd2-a7b0f5b1e9d8.vi/e85f0252-b661-475b-8e20-7d78206805a9.vi/805f8906-2ac2-4943-bcc2-ce7ee6626e70.vi/1a5fcff8-1e1b-4a10-8cb0-04266a3492f5.vi/1d7d714c-68c9-46d5-97e7-ece508b40457.vi
  1a7f9d96-89a5-4905-829b-2a4edb26e723.vi/1be28d80-beb7-4371-90e4-946dee281c8c.vi/29c07661-3584-43cb-8413-0ad855bf1dd6.vi/274c10cc-6877-4fb6-876e-52686d1825c0.vi/04a1345e-4259-4b92-a067-0273b67cbd8a.vi
  1a7f9d96-89a5-4905-829b-2a4edb26e723.vi/3a062081-cf3a-4e63-a10a-adcd83a17c12.vi/92de0394-8b0e-41a9-bbdb-0ba419639912.vi/ec3eeeb6-efa3-447e-bef4-ff225729b20e.vi/872e9e59-3680-4f22-9b9d-15434c4e78c9.vi
  1a7f9d96-89a5-4905-829b-2a4edb26e723.vi/70040952-3ae0-468b-bc38-5f997367fd6f.vi/85e2adf1-435c-4f2b-9704-a4fe5359d41d.vi/53a65439-65bc-4240-a9ef-cc811b2bd780.vi/2899dd3f-3718-40ac-92be-749708dd3abb.vi
  cfafe85d-2515-4c22-937f-8121ed6e9d54.vi/11fa2f37-74a1-4205-9996-7863193281ff.vi/e77d8312-4832-4633-a75f-e330979cf09b.vi/aed36081-aed2-409f-bc39-66819cd0b4c3.vi/3bf3b40a-782a-45e2-b8a0-653afe03bd13.vi
  cfafe85d-2515-4c22-937f-8121ed6e9d54.vi/07d86764-f698-4878-be38-d6e095ca1645.vi/c76a7bcb-882a-45a4-b89f-2597d2f33847.vi/54c288f8-840e-43b8-aaff-0bb173d43f54.vi/52b061ae-82a4-4929-86dd-60e1c67210a0.vi
  cfafe85d-2515-4c22-937f-8121ed6e9d54.vi/c0e3ea08-1ccb-4dcb-b733-8d3fe66c5f6f.vi/c3839c05-a494-4270-b8a7-0c53a6508c74.vi/3cadb2ed-87ca-4814-8e99-a2e720a8dfb1.vi/d5a0ec0b-00c1-4e11-af1d-53093ed117e4.vi
  LV2Julia_core/VIs/check ID validity.vi
  LV2Julia_core/VIs/bindata_descr to JSON.vi
  LV2Julia_core/VIs/check cluster field names.vi
  LV2Julia_core/VIs/concat JSON.vi
  LV2Julia_core/LV2Julia_core.lvlib
panel:
  out "arr dimension":i32
  out "numeric type":T1
  out "detailed error info":T2
  out "all elems OK":bool
  out "elem sent":cdb
  out "all arrays OK":bool
  in  "Stop JL-server":bool
  out "elem received":cdb
  out "numarray 3D":cdb[][][](array[numeric])
  out "numarray 2D":cdb[][](array[numeric])
  out "arrs equal":bool
  out "numarray 1D":cdb[](array[numeric]) format="%.1f"
  in  "index to return":cluster{"idx":u16[]}={"idx"=[1, 1, 1]} {"idx" min=1}
  out "Jl Server state out":T4
  out "short err code":u8
  out "final error":errorcluster
  # "add starting Jl server"
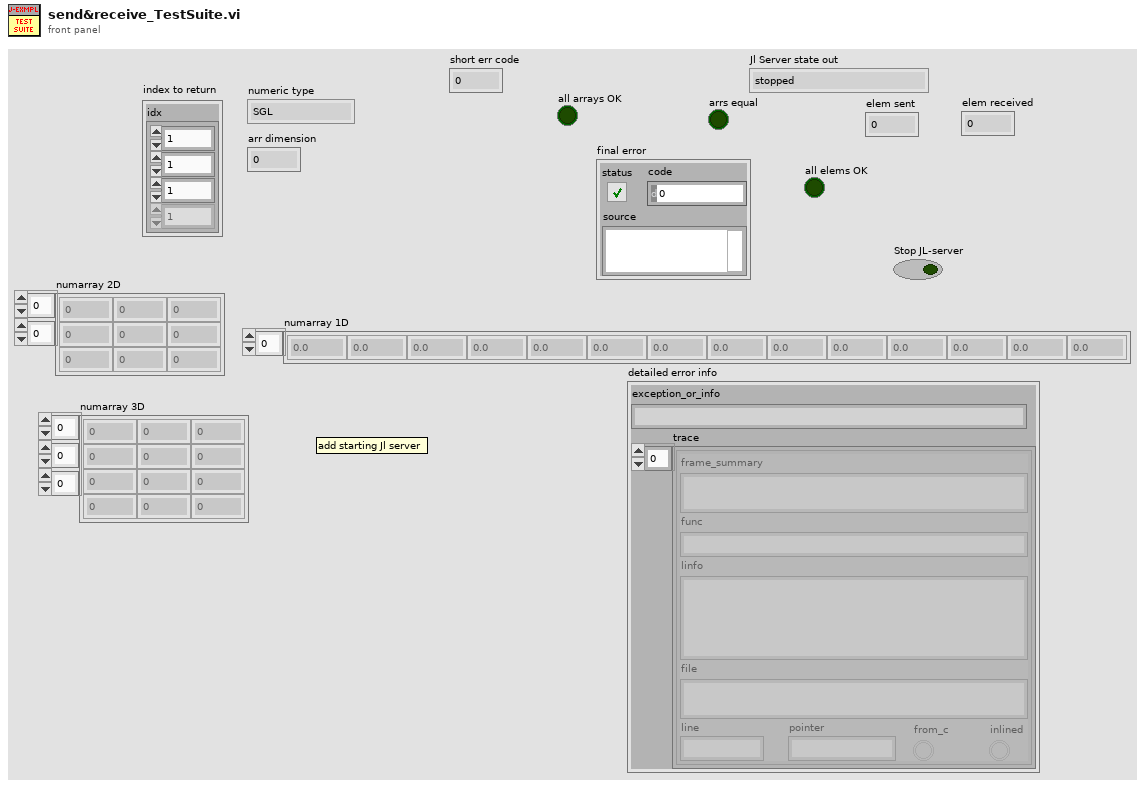
[diagram p1: front panel]
types:
  T1 = typedef "LV2Julia_core.lvlib/Numeric Types enum.ctl" = enum16{"SGL", "DBL", "I8", "I16", "I32", "I64", "U8", "U16", "U32", "U64", "CSGL", "CDBL", "boolean"}
  T2 = typedef "LV2Julia_core.lvlib/detailed error info.ctl" = cluster{"exception_or_info":string, "trace":T3[]}
  T3 = typedef "LV2Julia_core.lvlib/StackFrame.ctl" = cluster{"frame_summary":string, "func":string, "linfo":string, "file":string, "line":i32, "pointer":u64, "from_c":bool, "inlined":bool}
  T4 = typedef "LV2Julia_core.lvlib/Server or client state.ctl" = enum16{"stopped", "running", "unknown"}
  T5 = typedef "LV2Julia_core.lvlib/Commands.ctl" = enum16{"Start Jl-server & Init LV-client", "Send request & Get response ", "Stop Jl-server & Cleanup LV-client", "Cleanup LV-client", "Start Jl-server", "Stop Jl-server", "Init LV-Client", "Cleanup LV-Client", "(not allowed)", "Set LV Client state", "Set Jl Server state", "set ZMQ timeout", "read ZMQ timeout", "read-out state"}
  T6 = typedef "LV2Julia_core.lvlib/commands LV2Jl.ctl" = u8
  T7 = typedef "LV2Julia_core.lvlib/Bindata&description.ctl" = cluster{"bindata_descr":T8[], "bindata":u8[]}
  T8 = typedef "LV2Julia_core.lvlib/Bindata description.ctl" = cluster{"nofbytes":i32, "numtype":string, "start":i32, "arrdims":i32[], "kwarg_name":string, "category":string}
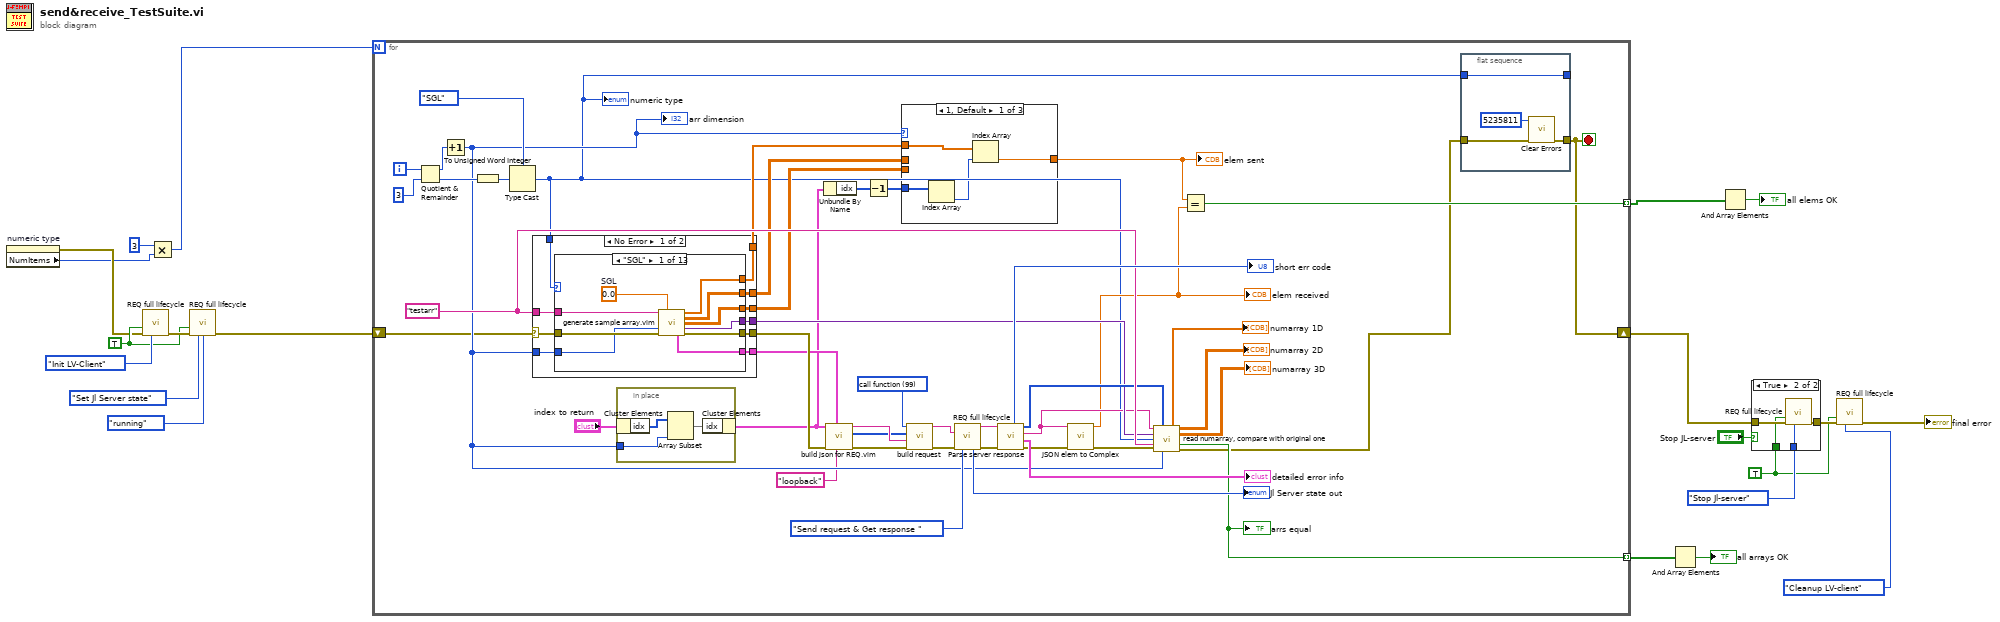
[diagram p0: block diagram]
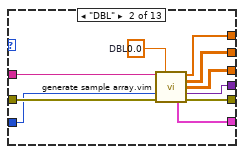
[diagram p2: hidden frame]
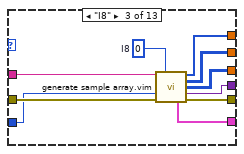
[diagram p3: hidden frame]
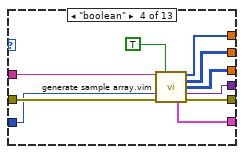
[diagram p4: hidden frame]
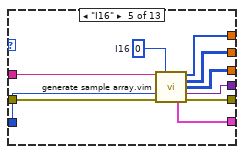
[diagram p5: hidden frame]
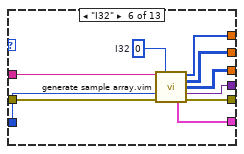
[diagram p6: hidden frame]
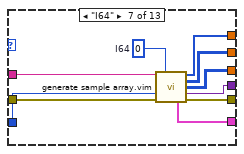
[diagram p7: hidden frame]
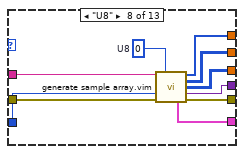
[diagram p8: hidden frame]
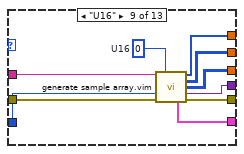
[diagram p9: hidden frame]
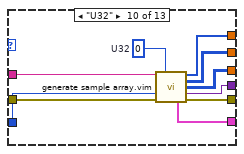
[diagram p10: hidden frame]
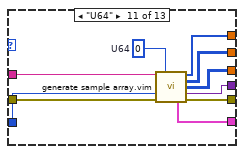
[diagram p11: hidden frame]
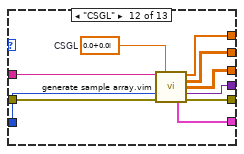
[diagram p12: hidden frame]
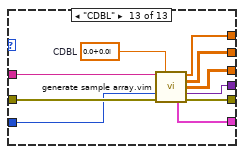
[diagram p13: hidden frame]
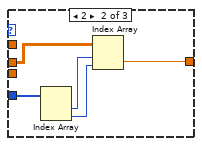
[diagram p15: hidden frame]
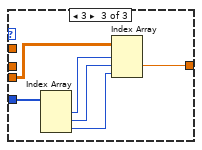
[diagram p16: hidden frame]
diagram:
  w12 = TRUE ("Force command")
  w16 = TRUE ("Force command")
  n1 = property on="numeric type" class="Enum (strict)"() -> (error out=w9:errorcluster, "NumItems"=w8:u32)  [unwired: 2 in, 1 out]
  n2 = call "REQ full lifecycle.vi"("Force command"=w12, "error in"=w9, "command"=Commands."Init LV-Client") -> ("error out"=w14:errorcluster)  [unwired: 6 in, 6 out]
  n3 = Multiply(x=u32 3, y=w8) -> (x*y=w6:u32)
  n4 = call "REQ full lifecycle.vi"("Force command"=w12, "error in"=w14, "command"=Commands."Set Jl Server state", "Jl Server state in"=Server_or_client_state."running") -> ("error out"=w3:errorcluster)  [unwired: 5 in, 6 out]
  n5 = for {
    N: w6 -> [_]
    tunnel: [w40] -> w5 mode=indexing
    shift-right: [w24] -> w21
    shift-left: w3 -> [w27]
    tunnel: [w29] -> w1 mode=indexing
    i -> [w44]
    stop <- w24 stop-if-true
    w53 = "testarr" ("Tag")
    w61 = T6 99 items=["call function"=99, "ping"=112, "stop"=115] ("Command")
    n6 = Quotient & Remainder(x=w44, y=3) -> (x-y*floor(x/y)=w36:i32, floor(x/y)=w38:i32)
    n7 = Increment(x=w36) -> (x+1=w28:i32)
    "arr dimension" <- w28
    n8 = To Unsigned Word Integer(number=w38) -> (unsigned 16bit integer=w41:u16)
    n9 = Type Cast(type=Numeric_Types_enum."SGL" ("numeric type const"), x=w41) -> (*(type *) &x=w25:T1)
    "numeric type" <- w25
    n10 = case shown="No Error" w27 {
      selector: w27 -> [w72 w212]
      tunnel: [w81 w212] -> w60
      tunnel: [w80 _] -> w59
      tunnel: w53 -> [w79 _]
      tunnel: [w78 _] -> w49
      tunnel: w25 -> [w77 _]
      tunnel: [w76 _] -> w35
      tunnel: [w75 _] -> w33
      tunnel: [w74 _] -> w32
      tunnel: w28 -> [w73 _]
      frame No Error {
        n11 = case shown="\"SGL\"" w77 {
          tunnel: [w91 w101 w111 w121 w131 w141 w151 w161 w171 w181 w191 w201 w211] -> w81
          tunnel: [w90 w100 w110 w120 w130 w140 w150 w160 w170 w180 w190 w200 w210] -> w80
          tunnel: w72 -> [w89 w99 w109 w119 w129 w139 w149 w159 w169 w179 w189 w199 w209]
          tunnel: w73 -> [w88 w98 w108 w118 w128 w138 w148 w158 w168 w178 w188 w198 w208]
          tunnel: w79 -> [w87 w97 w107 w117 w127 w137 w147 w157 w167 w177 w187 w197 w207]
          tunnel: [w85 w95 w105 w116 w125 w135 w145 w155 w165 w175 w185 w195 w205] -> w78
          tunnel: [w84 w92 w102 w113 w122 w132 w142 w152 w162 w172 w182 w192 w202] -> w74
          tunnel: [w83 w93 w103 w114 w123 w133 w143 w153 w163 w173 w183 w193 w203] -> w75
          tunnel: [w82 w94 w104 w115 w124 w134 w144 w154 w164 w174 w184 w194 w204] -> w76
          frame "SGL" {
            w86 = sgl 0.0  # SGL
            n12 = call "generate sample array.vim"("kwarg_name"=w87, "type"=w86, "dims"=w88, "error in (no error)"=w89) -> ("Array 1D"=w82:sgl[], "Array 2D"=w83:sgl[][], "Array 3D"=w84:sgl[][][], "array as variant"=w85:variant, "Bindata & descr out"=w90:T7, "error out"=w91:errorcluster)  [unwired: 5 in, 1 out]
          }
          frame "DBL" {
            w96 = 0.0  # DBL
            n13 = call "generate sample array.vim"("kwarg_name"=w97, "type"=w96, "dims"=w98, "error in (no error)"=w99) -> ("Array 1D"=w94:dbl[], "Array 2D"=w93:dbl[][], "Array 3D"=w92:dbl[][][], "array as variant"=w95:variant, "Bindata & descr out"=w100:T7, "error out"=w101:errorcluster)  [unwired: 5 in, 1 out]
          }
          frame "I8" {
            w106 = i8 0  # I8
            n14 = call "generate sample array.vim"("kwarg_name"=w107, "type"=w106, "dims"=w108, "error in (no error)"=w109) -> ("Array 1D"=w104:i8[], "Array 2D"=w103:i8[][], "Array 3D"=w102:i8[][][], "array as variant"=w105:variant, "Bindata & descr out"=w110:T7, "error out"=w111:errorcluster)  [unwired: 5 in, 1 out]
          }
          frame "boolean" {
            n15 = call "generate sample array.vim"("kwarg_name"=w117, "type"=TRUE, "dims"=w118, "error in (no error)"=w119) -> ("Array 1D"=w115:i16[], "Array 2D"=w114:i16[][], "Array 3D"=w113:i16[][][], "array as variant"=w116:variant, "Bindata & descr out"=w120:T7, "error out"=w121:errorcluster)  [unwired: 5 in, 1 out]
          }
          frame "I16" {
            w126 = i16 0  # I16
            n16 = call "generate sample array.vim"("kwarg_name"=w127, "type"=w126, "dims"=w128, "error in (no error)"=w129) -> ("Array 1D"=w124:i16[], "Array 2D"=w123:i16[][], "Array 3D"=w122:i16[][][], "array as variant"=w125:variant, "Bindata & descr out"=w130:T7, "error out"=w131:errorcluster)  [unwired: 5 in, 1 out]
          }
          frame "I32" {
            w136 = 0  # I32
            n17 = call "generate sample array.vim"("kwarg_name"=w137, "type"=w136, "dims"=w138, "error in (no error)"=w139) -> ("Array 1D"=w134:i32[], "Array 2D"=w133:i32[][], "Array 3D"=w132:i32[][][], "array as variant"=w135:variant, "Bindata & descr out"=w140:T7, "error out"=w141:errorcluster)  [unwired: 5 in, 1 out]
          }
          frame "I64" {
            w146 = i64 0  # I64
            n18 = call "generate sample array.vim"("kwarg_name"=w147, "type"=w146, "dims"=w148, "error in (no error)"=w149) -> ("Array 1D"=w144:i64[], "Array 2D"=w143:i64[][], "Array 3D"=w142:i64[][][], "array as variant"=w145:variant, "Bindata & descr out"=w150:T7, "error out"=w151:errorcluster)  [unwired: 5 in, 1 out]
          }
          frame "U8" {
            w156 = u8 0  # U8
            n19 = call "generate sample array.vim"("kwarg_name"=w157, "type"=w156, "dims"=w158, "error in (no error)"=w159) -> ("Array 1D"=w154:u8[], "Array 2D"=w153:u8[][], "Array 3D"=w152:u8[][][], "array as variant"=w155:variant, "Bindata & descr out"=w160:T7, "error out"=w161:errorcluster)  [unwired: 5 in, 1 out]
          }
          frame "U16" {
            w166 = u16 0  # U16
            n20 = call "generate sample array.vim"("kwarg_name"=w167, "type"=w166, "dims"=w168, "error in (no error)"=w169) -> ("Array 1D"=w164:u16[], "Array 2D"=w163:u16[][], "Array 3D"=w162:u16[][][], "array as variant"=w165:variant, "Bindata & descr out"=w170:T7, "error out"=w171:errorcluster)  [unwired: 5 in, 1 out]
          }
          frame "U32" {
            w176 = u32 0  # U32
            n21 = call "generate sample array.vim"("kwarg_name"=w177, "type"=w176, "dims"=w178, "error in (no error)"=w179) -> ("Array 1D"=w174:u32[], "Array 2D"=w173:u32[][], "Array 3D"=w172:u32[][][], "array as variant"=w175:variant, "Bindata & descr out"=w180:T7, "error out"=w181:errorcluster)  [unwired: 5 in, 1 out]
          }
          frame "U64" {
            w186 = u64 0  # U64
            n22 = call "generate sample array.vim"("kwarg_name"=w187, "type"=w186, "dims"=w188, "error in (no error)"=w189) -> ("Array 1D"=w184:u64[], "Array 2D"=w183:u64[][], "Array 3D"=w182:u64[][][], "array as variant"=w185:variant, "Bindata & descr out"=w190:T7, "error out"=w191:errorcluster)  [unwired: 5 in, 1 out]
          }
          frame "CSGL" {
            w196 = csg 0.0+0.0i  # CSGL
            n23 = call "generate sample array.vim"("kwarg_name"=w197, "type"=w196, "dims"=w198, "error in (no error)"=w199) -> ("Array 1D"=w194:csg[], "Array 2D"=w193:csg[][], "Array 3D"=w192:csg[][][], "array as variant"=w195:variant, "Bindata & descr out"=w200:T7, "error out"=w201:errorcluster)  [unwired: 5 in, 1 out]
          }
          frame "CDBL" {
            w206 = cdb 0.0+0.0i  # CDBL
            n24 = call "generate sample array.vim"("kwarg_name"=w207, "type"=w206, "dims"=w208, "error in (no error)"=w209) -> ("Array 1D"=w204:cdb[], "Array 2D"=w203:cdb[][], "Array 3D"=w202:cdb[][][], "array as variant"=w205:variant, "Bindata & descr out"=w210:T7, "error out"=w211:errorcluster)  [unwired: 5 in, 1 out]
          }
        }
      }
      frame Error {
      }
    }
    n25 = in-place {
      in-place-border: w28 -> [w229]
      n26 = in-place-cluster #1("index to return") -> ("idx"=w230:u16[])
      n27 = Array Subset(array=w230, length=w229) -> (w228:u16[])  [unwired: 1 in]
      n28 = in-place-cluster #1("idx"=w228) -> (w39:cluster{"idx":u16[]})
    }
    n29 = Unbundle By Name(w39) -> ("idx"=w37:u16[])
    n30 = call "build json for REQ.vim"("fun2call"="loopback", "Bindata & descr in"=w59, "error in (no error)"=w60, "Arguments 1"=w39) -> ("error out"=w66:errorcluster, "bindata out"=w55:u8[], "JSON string out"=w56:string)  [unwired: 5 in]
    n31 = Decrement(x=w37) -> (x-1=w34:u16[])
    n32 = case shown="1, Default" w28 {
      tunnel: w35 -> [w216 _ _]
      tunnel: w34 -> [w215 w221 w227]
      tunnel: [w213 w219 w225] -> w31
      tunnel: w33 -> [_ w218 _]
      tunnel: w32 -> [_ _ w223]
      frame 1, Default {
        n33 = Index Array(array=w215) -> (element=w214:u16)  [unwired: 1 in]
        n34 = Index Array(array=w216, index=w214) -> (element=w213:cdb)
      }
      frame 2 {
        n35 = Index Array(array=w221) -> (element #1=w220:u16, element #2=w217:u16)  [unwired: 2 in]
        n36 = Index Array(array=w218, index (row)=w220, index (col)=w217) -> (element=w219:cdb)
      }
      frame 3 {
        n37 = Index Array(array=w227) -> (element #1=w226:u16, element #2=w224:u16, element #3=w222:u16)  [unwired: 3 in]
        n38 = Index Array(array=w223, index (dim 0)=w226, index (dim 1)=w224, index (dim 2)=w222) -> (element=w225:cdb)
      }
    }
    "elem sent" <- w31
    n39 = call "build request.vi"("error in (no error)"=w66, "JSON data"=w56, "binary data"=w55, "Command"=w61) -> ("error out"=w64:errorcluster, "REQ string"=w65:string)  [unwired: 6 in]
    n40 = call "REQ full lifecycle.vi"("data to send"=w65, "error in"=w64, "command"=Commands."Send request & Get response ") -> ("server response"=w22:string, "Jl Server state out"=→"Jl Server state out":T4, "error out"=w63:errorcluster)  [unwired: 6 in, 4 out]
    n41 = call "Parse server response.vi"("error in (no error)"=w63, "server response in"=w22) -> ("error out"=w47:errorcluster, "detailed error info"=→"detailed error info":T2, "JSON out"=w45:string, "binary data"=w52:u8[], "return code"=→"short err code":u8)  [unwired: 2 in, 3 out]
    n42 = call "JSON elem to Complex.vi"("error in (no error)"=w47, "JSON in"=w45) -> ("error out"=w46:errorcluster, "Numeric"=w30:cdb)  [unwired: 8 in]
    "elem received" <- w30
    n43 = call "read numarray, compare with original one.vi"("JSON in"=w45, "binary data in"=w52, "array as variant in"=w49, "numeric type"=w25, "kwarg_name"=w53, "error in (no error)"=w46, "dims"=w28) -> ("numarray 1D"=→"numarray 1D":cdb[], "numarray 2D"=→"numarray 2D":cdb[][], "numarray 3D"=→"numarray 3D":cdb[][][], "arrays are equal"=w40:bool, "error out"=w26:errorcluster)  [unwired: 1 in, 3 out]
    "arrs equal" <- w40
    n44 = Equal?(x=w31, y=w30) -> (x = y?=w29:bool)
    n45 = flat-sequence {
      tunnel: w26 -> [w71]
      tunnel: [w70] -> w24
      tunnel: [w68] -> _
      tunnel: w25 -> [w68]
      frame #0 {
        n46 = call <vilib>:"Clear Errors.vi"("error in (no error)"=w71, "specific error code to clear (0: all)"=5235811) -> ("error out"=w70:errorcluster)  [unwired: 4 in, 1 out]
      }
    }
  }
  n47 = And Array Elements(Boolean array=w5) -> (logical AND=→"all arrays OK":bool)
  n48 = And Array Elements(Boolean array=w1) -> (logical AND=→"all elems OK":bool)
  n49 = case shown="True" "Stop JL-server" {
    tunnel: w21 -> [w231 w235]
    tunnel: Commands."Stop Jl-server" ("command") -> [_ w234]
    tunnel: [w231 w233] -> w19
    tunnel: w16 -> [_ w232]
    frame False {
    }
    frame True {
      n50 = call "REQ full lifecycle.vi"("Force command"=w232, "error in"=w235, "command"=w234) -> ("error out"=w233:errorcluster)  [unwired: 6 in, 6 out]
    }
  }
  n51 = call "REQ full lifecycle.vi"("Force command"=w16, "error in"=w19, "command"=Commands."Cleanup LV-client") -> ("error out"=→"final error":errorcluster)  [unwired: 6 in, 6 out]
